vi "Joystick and Camera SHIH VP- external Connection.vi"(0 "Motion in":refnum<class "Motion.lvclass">, 1 "XYZTheta":dbl[](array[numeric]), 2 "Measurement Point":string, 3 "Inital GO":bool=TRUE) -> (7 "Motion out":refnum<class "Motion.lvclass">, 8 "Sum":dbl[](array[numeric]), 9 "Gantry":dbl[](array[numeric]), 10 "error out":errorcluster)   [LabVIEW 2016]
uses:
  Classes/Controllers/Motion/Copy of Motion Folder/Motion.lvclass
  Classes/Controllers/Camera/Copy of Camera Folder/Machine Vision.ctl
  Classes/Controllers/Camera/Copy of Camera Folder/Camera.lvclass
  Classes/Controllers/Camera/Copy of Controller Folder/Controller.lvclass
panel:
  in  "change move step":bool
  in  "step":dbl=15.0
  in  "Z go up":bool
  in  "Z go down":bool
  in  "Machine Vision":T1
  in  "object goes left":bool
  in  "object goes right":bool
  in  "object goes down":bool
  in  "object goes up":bool
  in  "Z go up 25 um":bool
  in  "Z go down 25 um":bool
  in  "Z go up 0.05 mm":bool
  in  "Z go down 0.05 mm":bool
  in  "Z go  up 0.1 mm":bool
  in  "Z go down 0.1 mm":bool
  in  "Machine Vision 2":T1=enum."None"
  out "Image 2":T2(plugin-control)
  out "Focus Index":dbl[](array[numeric])
  in  "interval":dbl=0.005
  out "Score":dbl[](array[numeric])
  out "Waveform Graph":dbl[](graph)
  in  "focus":bool
  out "Numeric":dbl
  in  "Go SUM":bool
  in  "Z Go":bool
  in  "Position":dbl
  in  "Go":bool
  in  "Joystick":bool
  in  "Stop":bool
  out "Image":T2(plugin-control)
  out "Camera":dbl[](array[numeric])
  # "0.1mm"
  # "0.01mm"
  # "um"
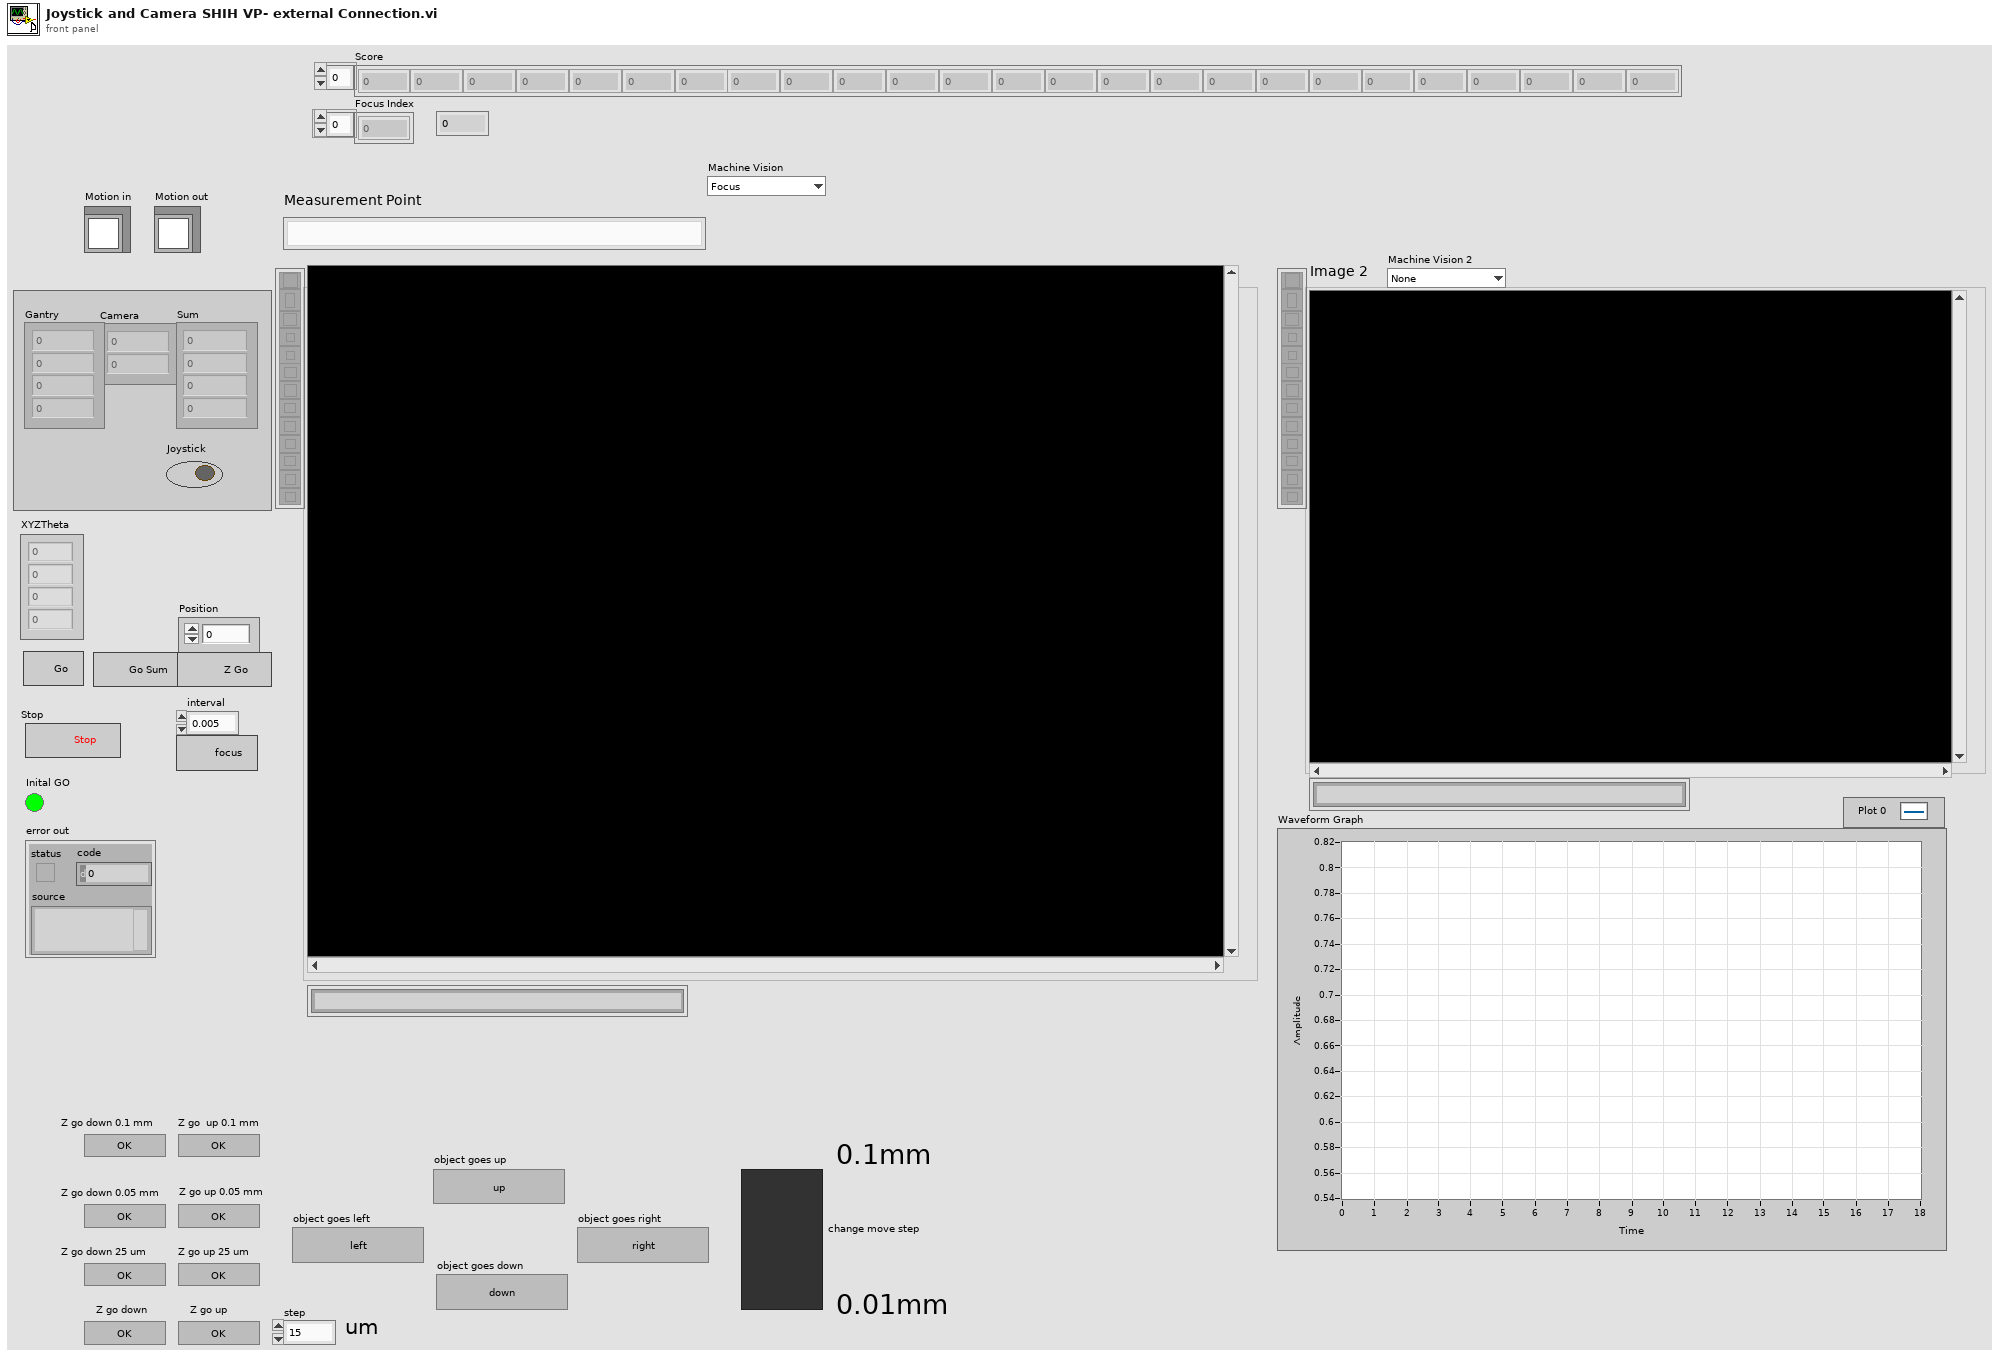
[diagram p1: front panel]
types:
  T1 = typedef "Camera.lvclass/Machine Vision.ctl" = enum16{"Focus", "chip cross", "LargeCircle", "None", "INTT HDI Mark", "INTT Sensor Cross", "INTT Chip Corner", "HPK Silicon", "circle"}
  T2 = typedef "IMAQ Image.ctl" = refnum<image>
  T3 = typedef "Controller.lvclass/Controllers.ctl" = cluster{"Copy of Motion.lvclass":refnum<class "Motion.lvclass">, "Copy of I-O.lvclass":refnum<class "I-O.lvclass">, "Copy of Dispenser.lvclass":refnum<class "Dispenser.lvclass">}
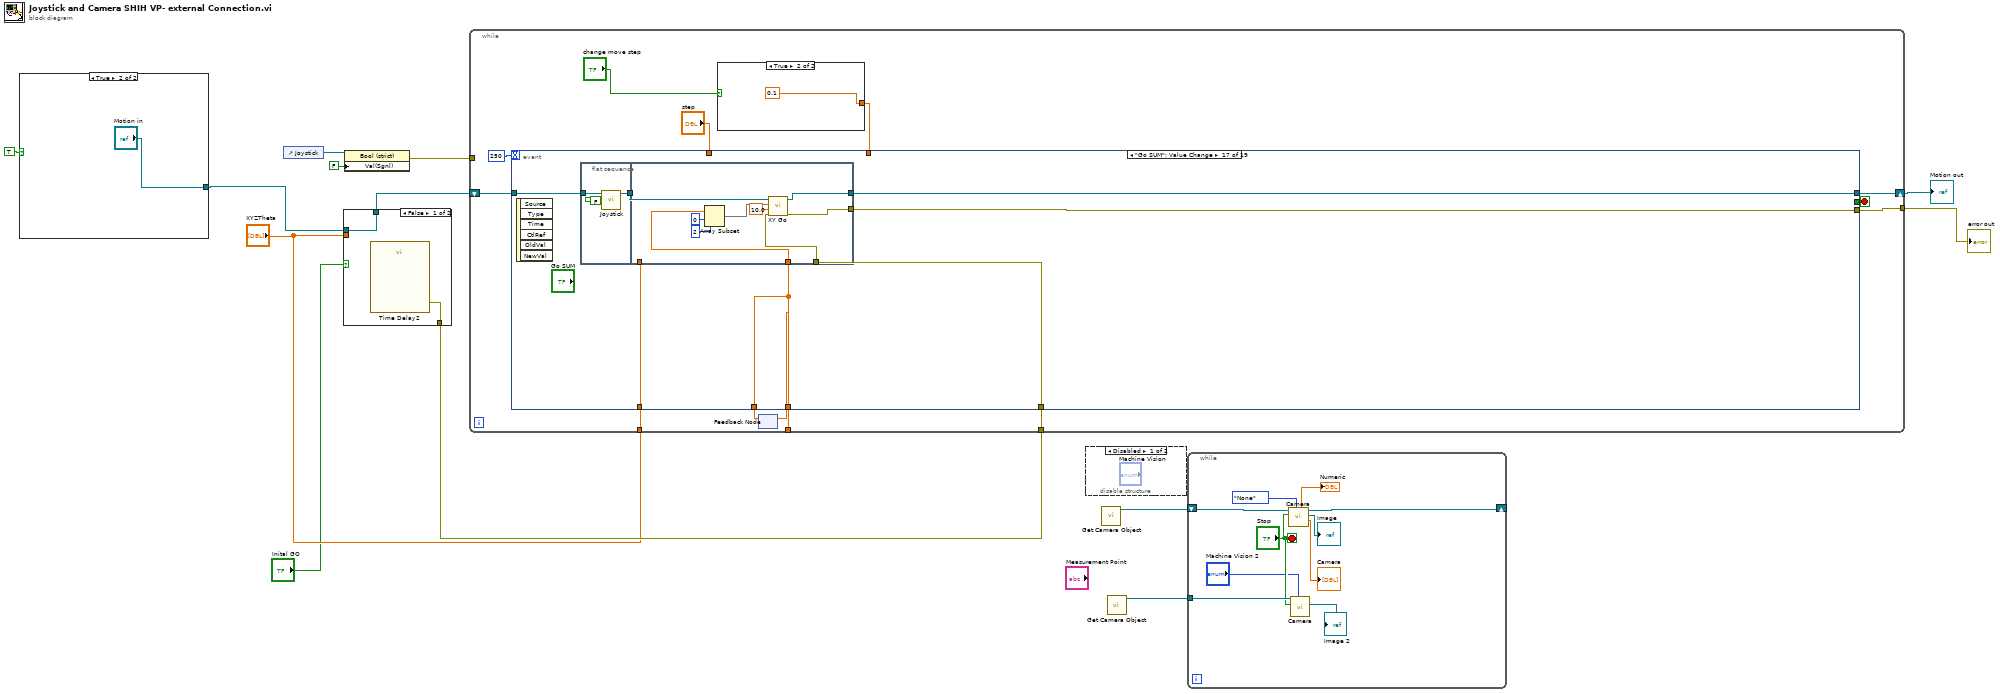
[diagram p0: block diagram]
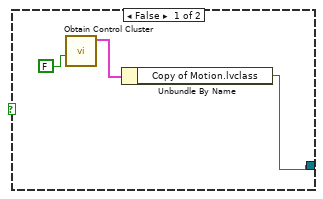
[diagram p3: hidden frame]
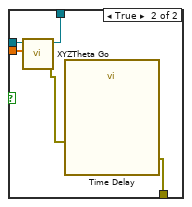
[diagram p4: hidden frame]
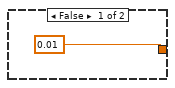
[diagram p5: hidden frame]
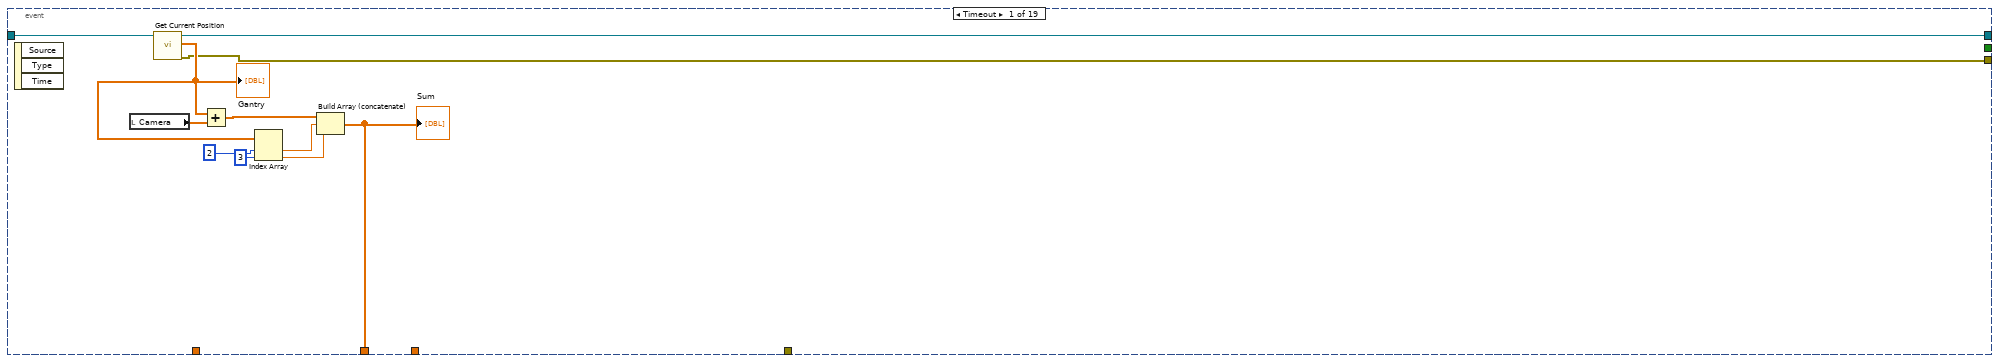
[diagram p6: hidden frame]
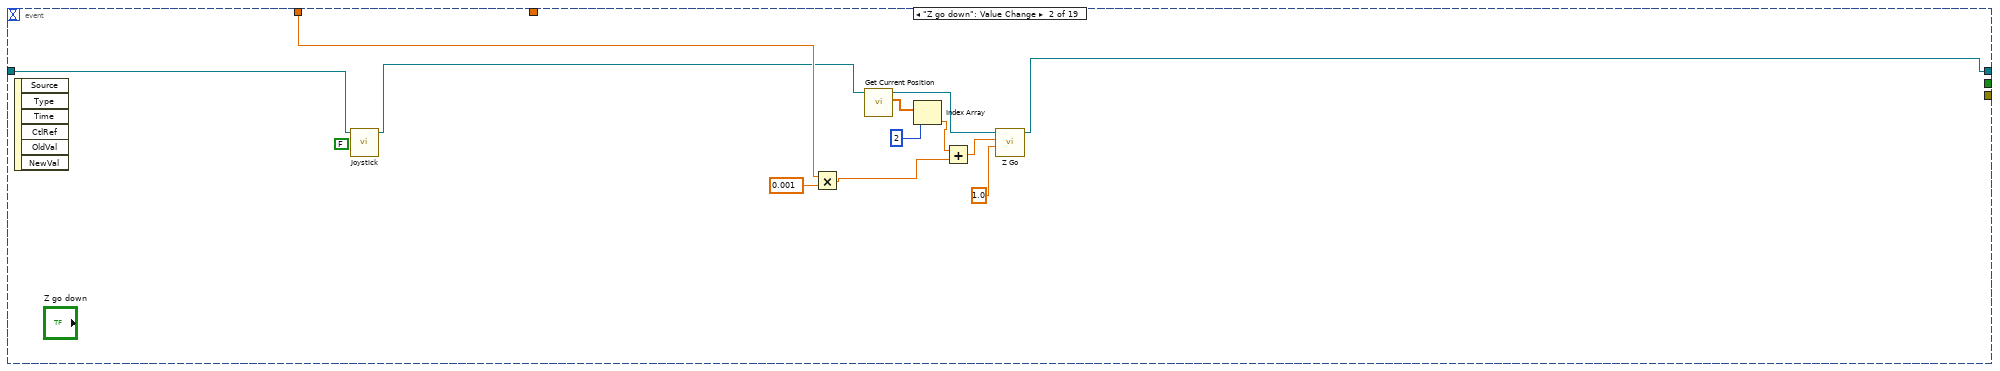
[diagram p7: hidden frame]
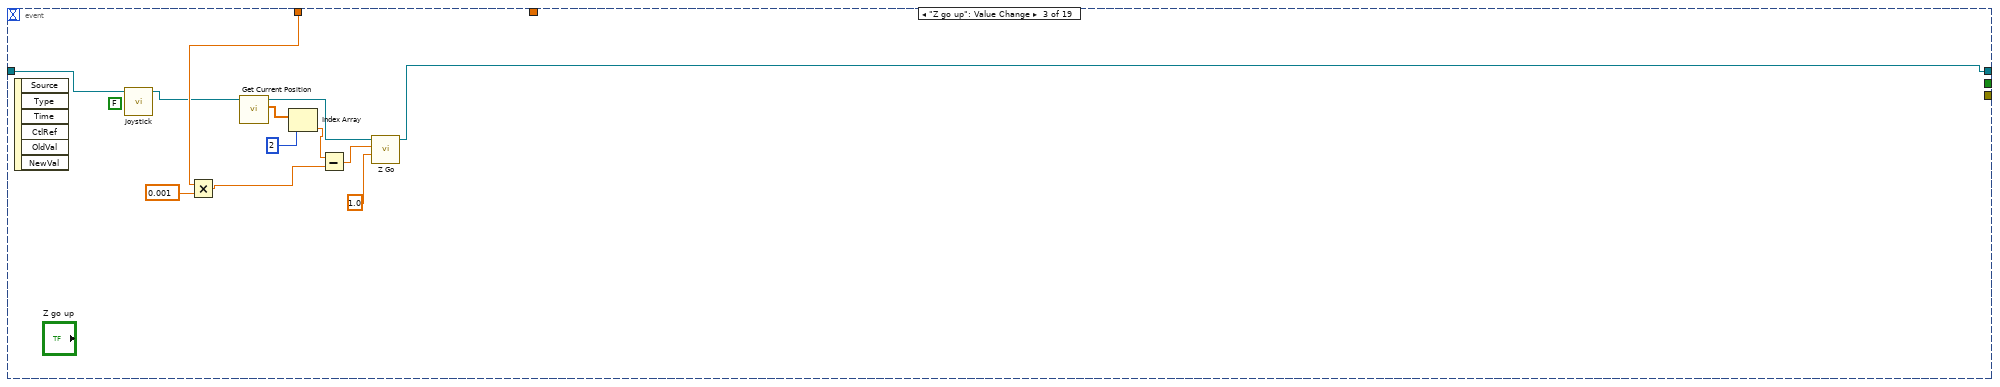
[diagram p8: hidden frame]
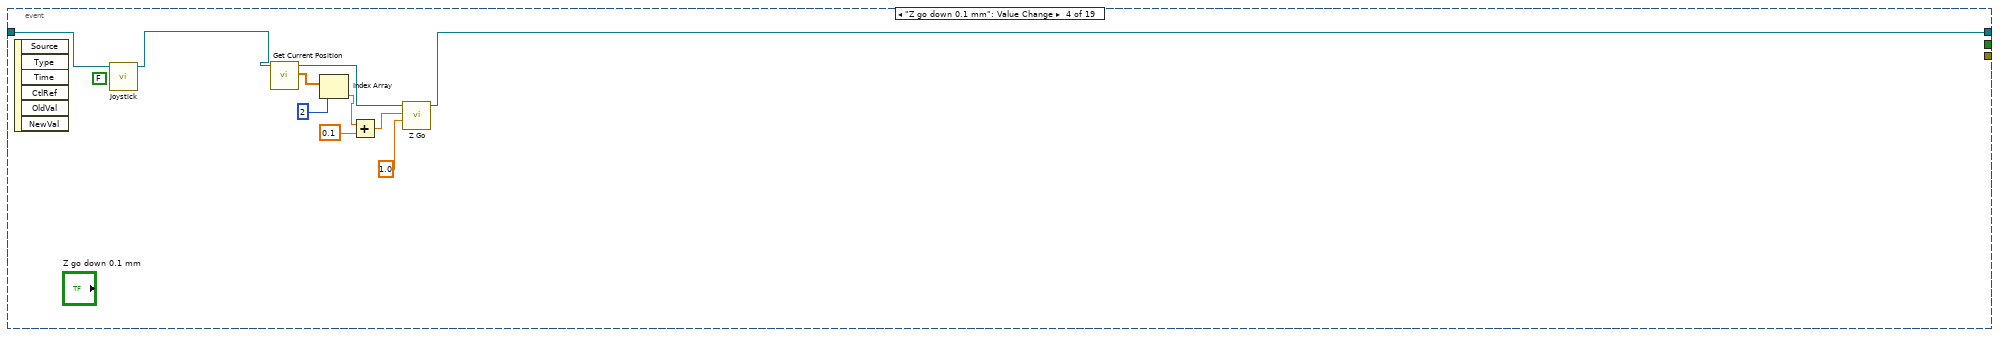
[diagram p9: hidden frame]
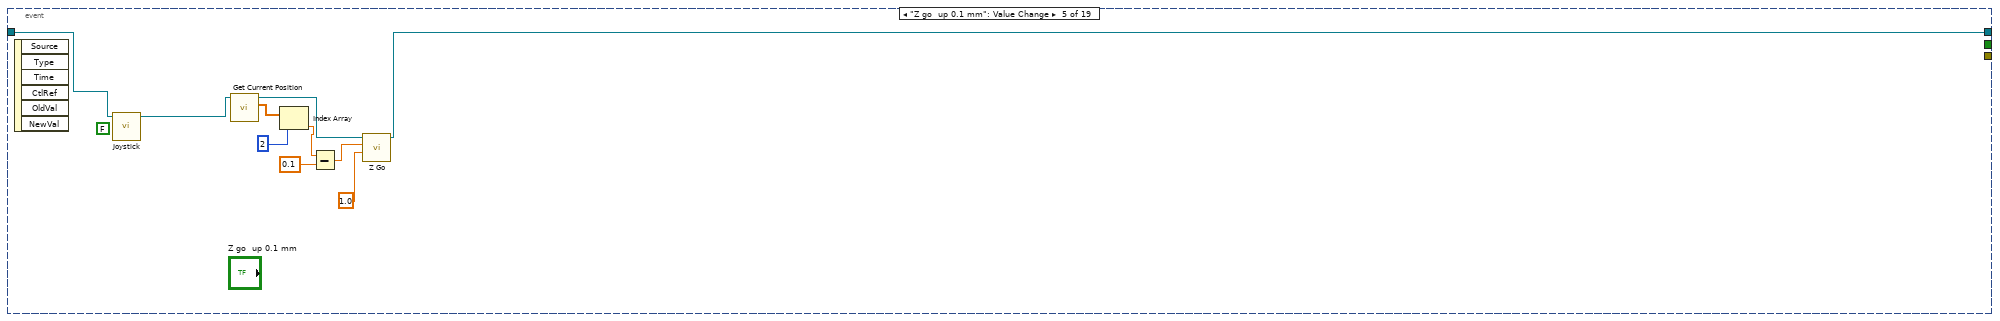
[diagram p10: hidden frame]
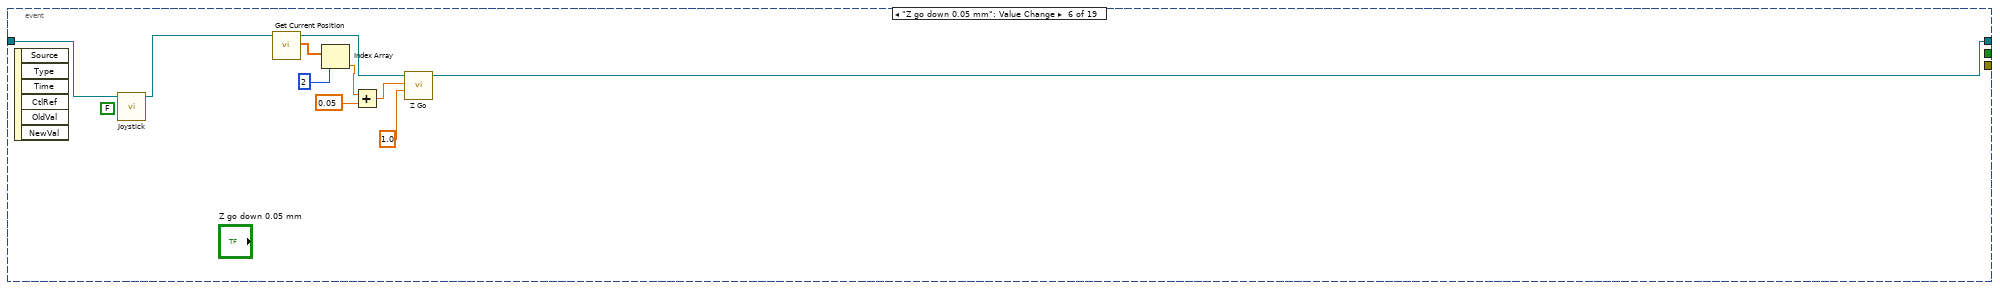
[diagram p11: hidden frame]
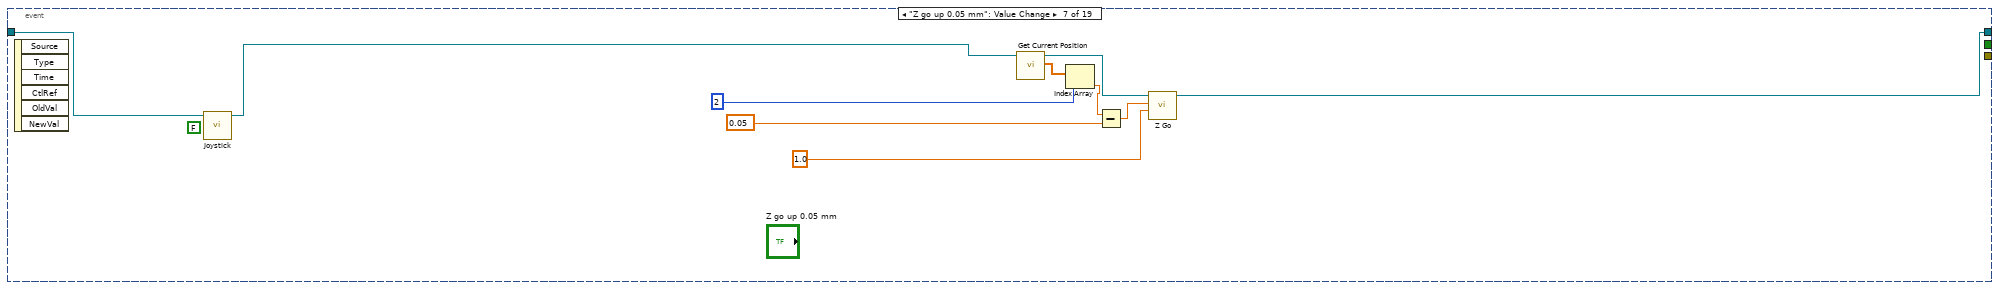
[diagram p12: hidden frame]
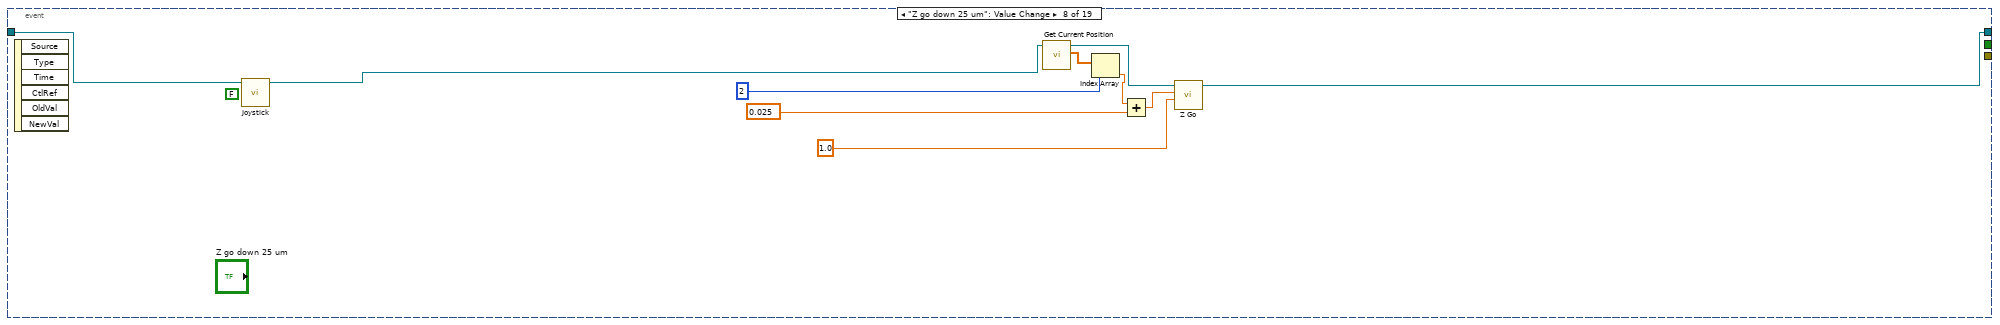
[diagram p13: hidden frame]
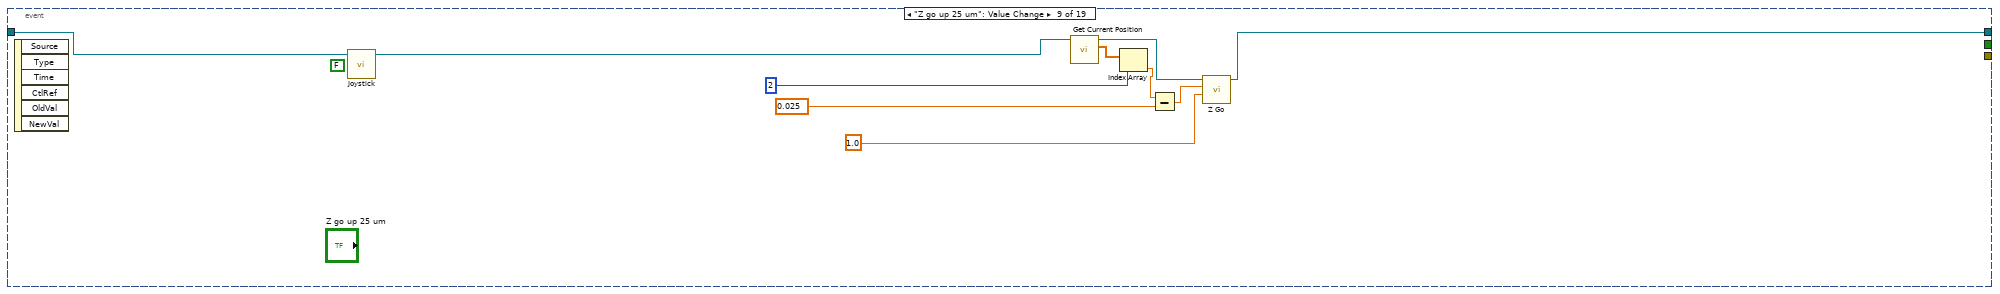
[diagram p14: hidden frame]
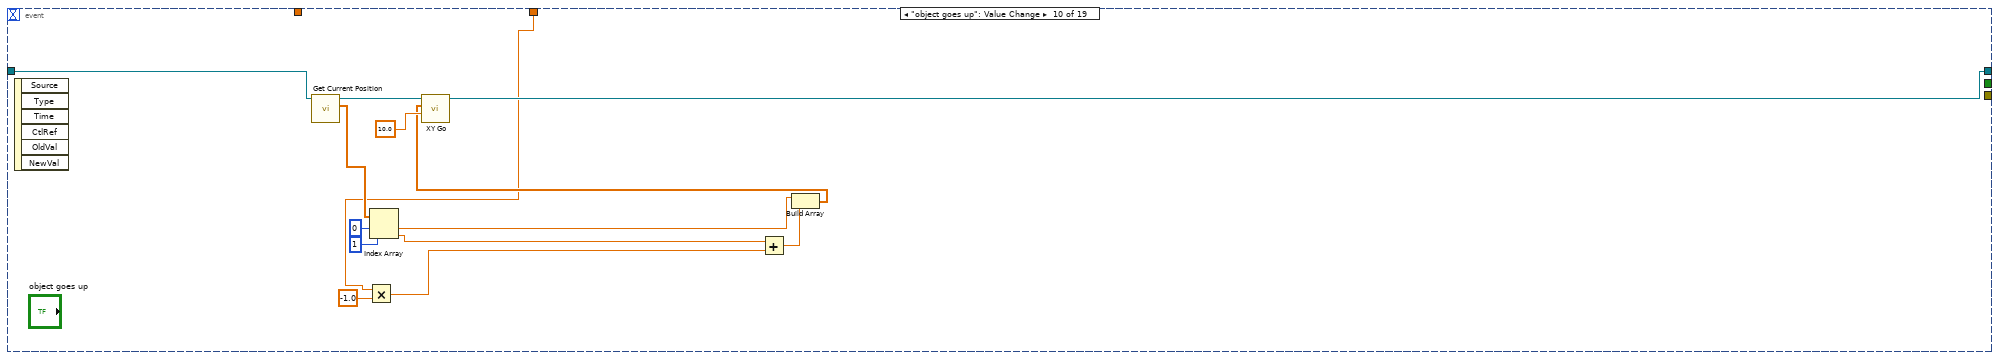
[diagram p15: hidden frame]
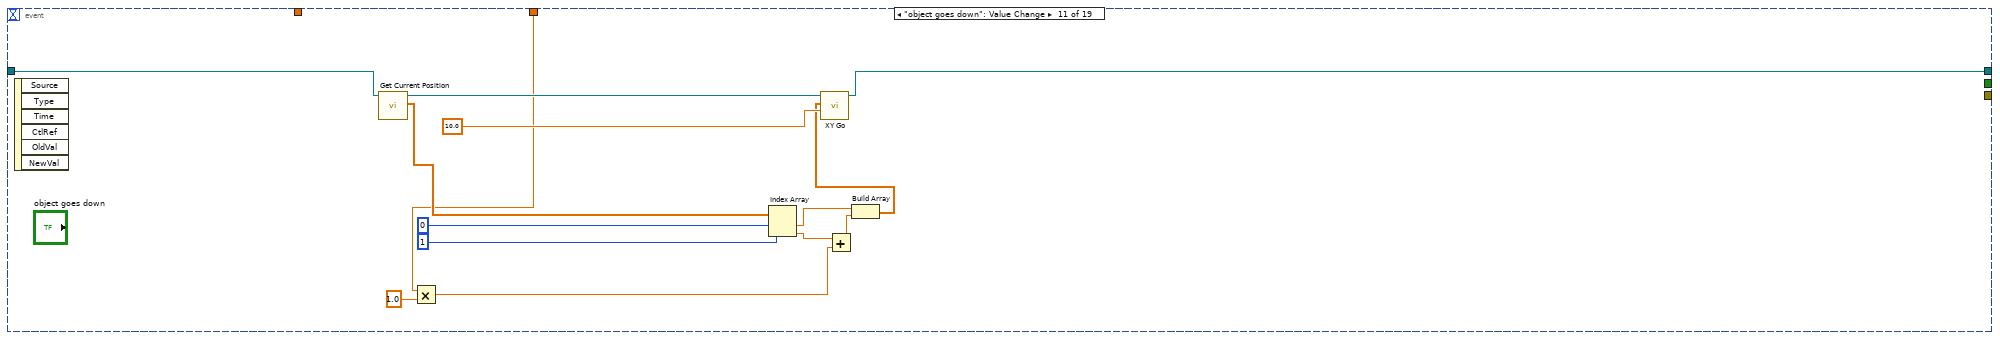
[diagram p16: hidden frame]
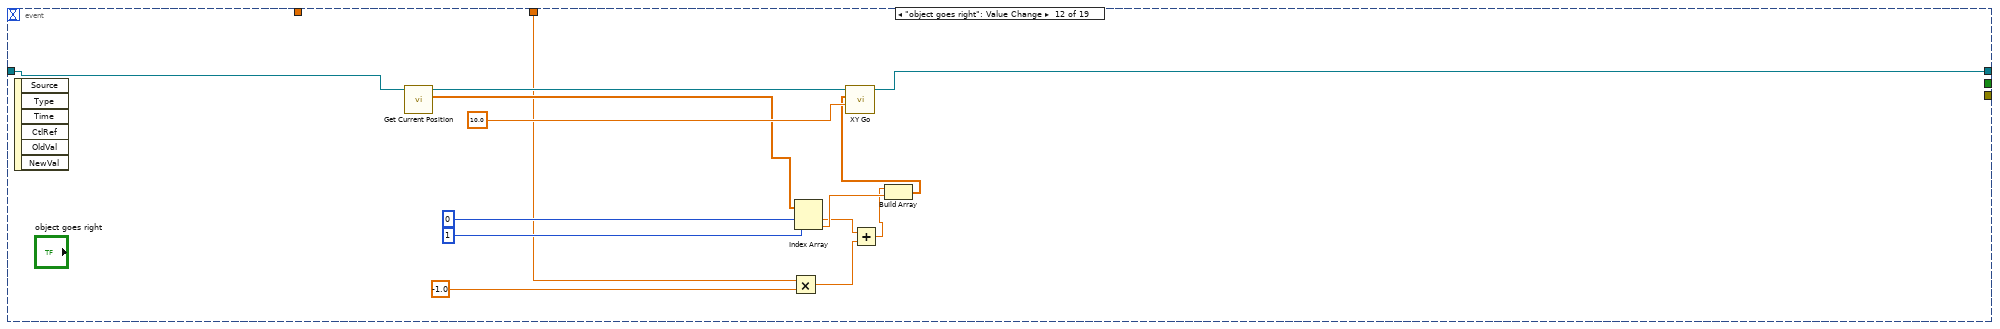
[diagram p17: hidden frame]
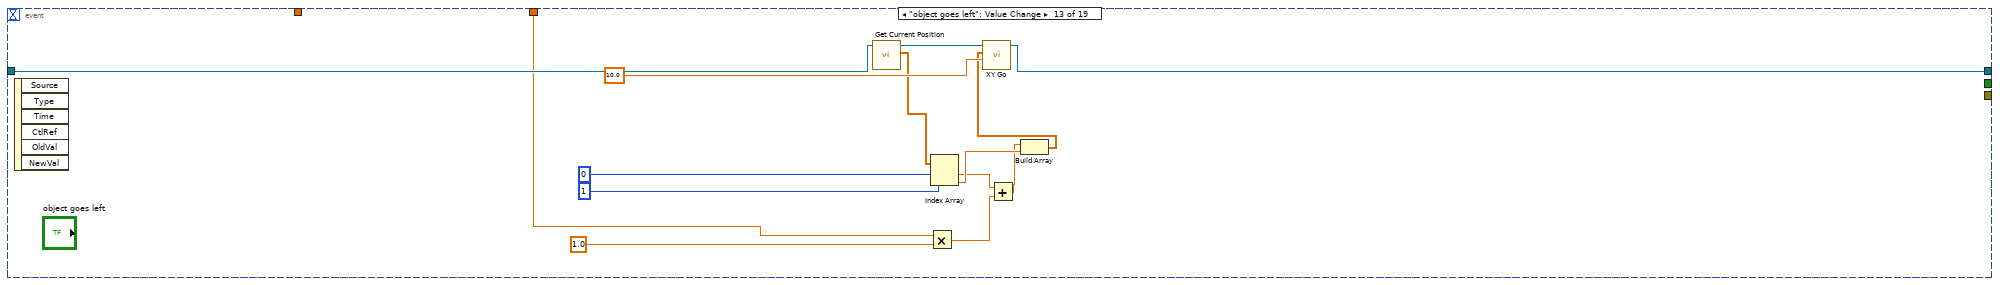
[diagram p18: hidden frame]
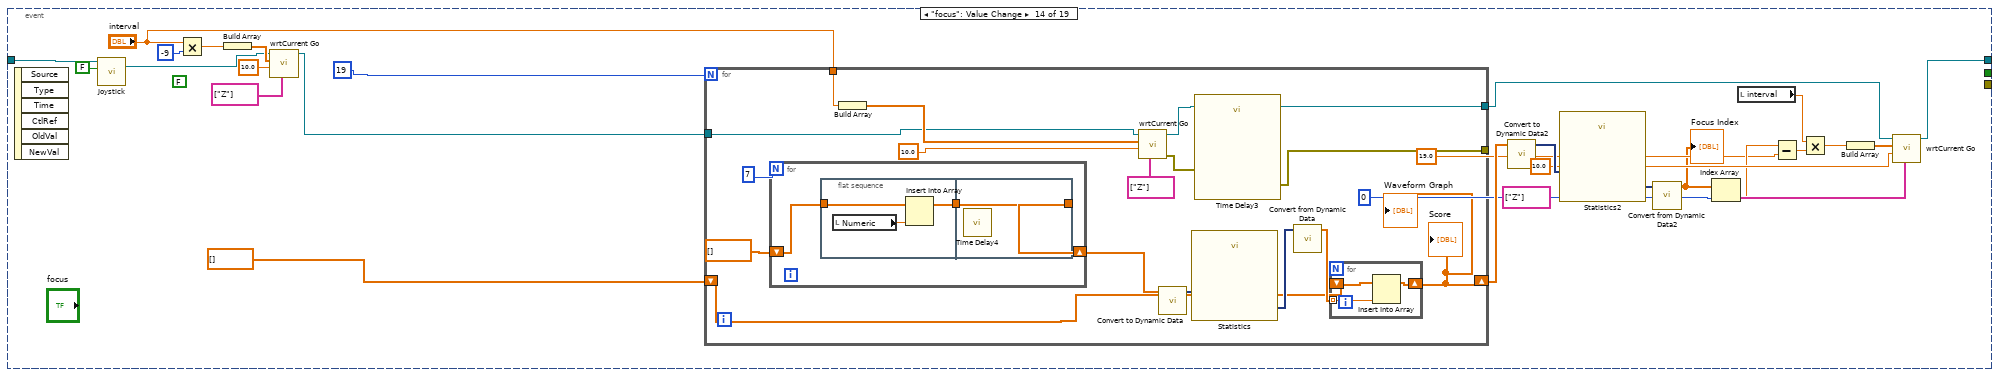
[diagram p19: hidden frame]
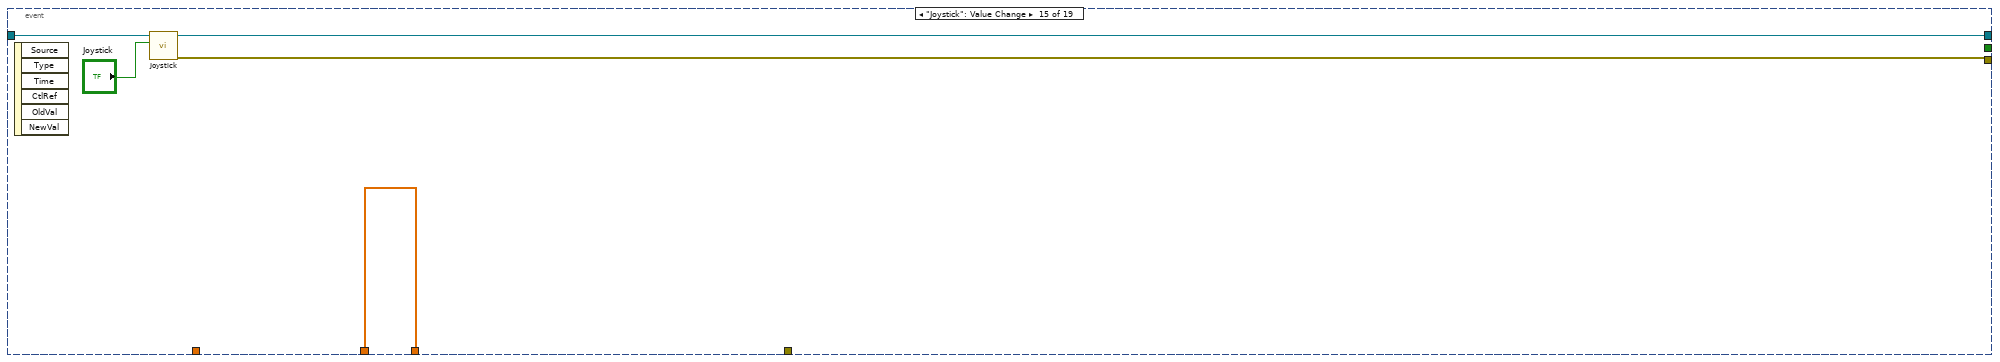
[diagram p20: hidden frame]
diagram:
  n1 = case shown="True" TRUE {
    tunnel: [w14 "Motion in"] -> w1
    frame False {
      n2 = call "Obtain Control Cluster.vi"("I/O"=FALSE) -> ("Control Out"=w16:T3)  [unwired: 10 in]
      n3 = Unbundle By Name(w16) -> ("Copy of Motion.lvclass"=w14:refnum<class "Motion.lvclass">)
    }
    frame True {
    }
  }
  n4 = control-ref of="Joystick"() -> (w12:refnum<vi>)
  n5 = case shown="False" "Inital GO" {
    tunnel: w1 -> [w19 w24]
    tunnel: [w19 w23] -> w7
    tunnel: [w18 w21] -> w6
    tunnel: "XYZTheta" -> [_ w20]
    frame False {
      n6 = call "Time Delay2"() -> ("error out"=w18:errorcluster)  [unwired: 11 in]
    }
    frame True {
      n7 = call "XYZTheta Go.vi"("XYZTheta In"=w20, "Motion in"=w24) -> ("error out"=w22:errorcluster, "Motion out"=w23:refnum<class "Motion.lvclass">)  [unwired: 7 in, 1 out]
      n8 = call "Time Delay"("error in (no error)"=w22) -> ("error out"=w21:errorcluster)  [unwired: 10 in]
    }
  }
  n9 = property class="Bool (strict)"(reference=w12, "Val(Sgnl)"=FALSE ("Value (Signaling)")) -> (error out=w11:errorcluster)  [unwired: 1 in, 1 out]
  n10 = while {
    shift-right: [w33] -> w9
    shift-left: w7 -> [w34]
    tunnel: w11 -> [_]
    tunnel: [w32] -> w8
    tunnel: w6 -> [w31]
    tunnel: "XYZTheta" -> [w30]
    tunnel: [w28] -> _
    stop <- w35 stop-if-true
    n11 = case shown="True" "change move step" {
      tunnel: [0.01 0.1] -> w25
      frame False {
      }
      frame True {
      }
    }
    n12 = feedback #1() -> (w28:dbl[])  [unwired: 1 in]
    n13 = event shown="[16] \"Go SUM\": Value Change" {
      selector: _ -> [_ _ _ _ _ _ _ _ _ _ _ _ _ _ _ _ _ _ _]
      dyn-events: _ -> [_ _ _ _ _ _ _ _ _ _ _ _ _ _ _ _ _ _ _]
      timeout: 250 -> [_ _ _ _ _ _ _ _ _ _ _ _ _ _ _ _ _ _ _]
      tunnel: [_ _ _ _ _ _ _ _ _ _ _ _ _ _ _ _ _ _ TRUE] -> w35
      tunnel: w34 -> [w48 w51 w63 w75 w85 w95 w105 w115 w125 w145 w155 w166 w180 w192 w247 w254 w279 w298 w302]
      tunnel: [w47 w52 w67 w76 w86 w96 w106 w116 w126 w144 w154 w167 w181 w191 w245 w253 w274 w297 w300] -> w33
      tunnel: [w42 _ _ _ _ _ _ _ _ _ _ _ _ _ w244 w251 w277 w292 _] -> w32
      tunnel: w31 -> [_ _ _ _ _ _ _ _ _ _ _ _ _ _ _ w250 w276 w293 _]
      tunnel: w30 -> [_ _ _ _ _ _ _ _ _ _ _ _ _ _ _ w249 w275 _ _]
      tunnel: [w39 _ _ _ _ _ _ _ _ _ _ _ _ _ w243 w248 w273 w294 w299] -> w29
      tunnel: w28 -> [_ _ _ _ _ _ _ _ _ _ _ _ _ _ w243 w248 w273 w294 w299]
      tunnel: "step" -> [_ w53 w65 _ _ _ _ _ _ _ _ _ _ _ _ _ _ _ _]
      tunnel: w25 -> [_ _ _ _ _ _ _ _ _ w134 w148 w162 w176 _ _ _ _ _ _]
      event Timeout {
        n14 = event-data() -> ()  [unwired: 1 in, 3 out]
        n15 = local read "Camera"() -> (w49:dbl[])
        n16 = call-dynamic "Get Current Position.vi"("Motion in"=w48) -> ("error out"=w42:errorcluster, "XYZTheta Out"=w45:dbl[], "Motion out"=w47:refnum<class "Motion.lvclass">)  [unwired: 8 in]
        "Gantry" <- w45
        n17 = Add(x=w45, y=w49) -> (x+y=w46:dbl[])
        n18 = Index Array(array=w45, index #1=2 ("index"), index #2=3 ("index")) -> (element #1=w43:dbl, element #2=w40:dbl)
        n19 = Build Array (concatenate)(w46, w43, w40) -> (w39:dbl[])
        "Sum" <- w39
      }
      event "Z go down": Value Change {
        (unwired) FALSE ("Joystick")
        n20 = event-data() -> ()  [unwired: 1 in, 6 out]
        n21 = call-dynamic "Joystick.vi"("Motion in"=w51) -> ("Motion out"=w50:refnum<class "Motion.lvclass">)  [unwired: 9 in, 1 out]
        n22 = Multiply(x=w53, y=0.001) -> (x*y=w55:dbl)
        n23 = call-dynamic "Get Current Position.vi"("Motion in"=w50) -> ("XYZTheta Out"=w61:dbl[], "Motion out"=w59:refnum<class "Motion.lvclass">)  [unwired: 8 in, 1 out]
        n24 = Index Array(array=w61, index=2) -> (element=w56:dbl)
        n25 = Add(x=w56, y=w55) -> (x+y=w57:dbl)
        n26 = call-dynamic "Z Go.vi"("Speed"=1.0, "Position"=w57, "Motion in"=w59) -> ("Motion out"=w52:refnum<class "Motion.lvclass">)  [unwired: 7 in, 1 out]
      }
      event "Z go up": Value Change {
        (unwired) FALSE ("Joystick")
        n27 = event-data() -> ()  [unwired: 1 in, 6 out]
        n28 = call-dynamic "Joystick.vi"("Motion in"=w63) -> ("Motion out"=w62:refnum<class "Motion.lvclass">)  [unwired: 9 in, 1 out]
        n29 = Multiply(x=w65, y=0.001) -> (x*y=w66:dbl)
        n30 = call-dynamic "Get Current Position.vi"("Motion in"=w62) -> ("XYZTheta Out"=w73:dbl[], "Motion out"=w71:refnum<class "Motion.lvclass">)  [unwired: 8 in, 1 out]
        n31 = Index Array(array=w73, index=2) -> (element=w68:dbl)
        n32 = Subtract(x=w68, y=w66) -> (x-y=w69:dbl)
        n33 = call-dynamic "Z Go.vi"("Speed"=1.0, "Position"=w69, "Motion in"=w71) -> ("Motion out"=w67:refnum<class "Motion.lvclass">)  [unwired: 7 in, 1 out]
      }
      event "Z go down 0.1 mm": Value Change {
        (unwired) FALSE ("Joystick")
        n34 = event-data() -> ()  [unwired: 1 in, 6 out]
        n35 = call-dynamic "Joystick.vi"("Motion in"=w75) -> ("Motion out"=w74:refnum<class "Motion.lvclass">)  [unwired: 9 in, 1 out]
        n36 = call-dynamic "Get Current Position.vi"("Motion in"=w74) -> ("XYZTheta Out"=w83:dbl[], "Motion out"=w81:refnum<class "Motion.lvclass">)  [unwired: 8 in, 1 out]
        n37 = Index Array(array=w83, index=2) -> (element=w78:dbl)
        n38 = Add(x=w78, y=0.1) -> (x+y=w79:dbl)
        n39 = call-dynamic "Z Go.vi"("Speed"=1.0, "Position"=w79, "Motion in"=w81) -> ("Motion out"=w76:refnum<class "Motion.lvclass">)  [unwired: 7 in, 1 out]
      }
      event "Z go  up 0.1 mm": Value Change {
        (unwired) FALSE ("Joystick")
        n40 = event-data() -> ()  [unwired: 1 in, 6 out]
        n41 = call-dynamic "Joystick.vi"("Motion in"=w85) -> ("Motion out"=w84:refnum<class "Motion.lvclass">)  [unwired: 9 in, 1 out]
        n42 = call-dynamic "Get Current Position.vi"("Motion in"=w84) -> ("XYZTheta Out"=w93:dbl[], "Motion out"=w91:refnum<class "Motion.lvclass">)  [unwired: 8 in, 1 out]
        n43 = Index Array(array=w93, index=2) -> (element=w88:dbl)
        n44 = Subtract(x=w88, y=0.1) -> (x-y=w89:dbl)
        n45 = call-dynamic "Z Go.vi"("Speed"=1.0, "Position"=w89, "Motion in"=w91) -> ("Motion out"=w86:refnum<class "Motion.lvclass">)  [unwired: 7 in, 1 out]
      }
      event "Z go down 0.05 mm": Value Change {
        (unwired) FALSE ("Joystick")
        n46 = event-data() -> ()  [unwired: 1 in, 6 out]
        n47 = call-dynamic "Joystick.vi"("Motion in"=w95) -> ("Motion out"=w94:refnum<class "Motion.lvclass">)  [unwired: 9 in, 1 out]
        n48 = call-dynamic "Get Current Position.vi"("Motion in"=w94) -> ("XYZTheta Out"=w103:dbl[], "Motion out"=w101:refnum<class "Motion.lvclass">)  [unwired: 8 in, 1 out]
        n49 = Index Array(array=w103, index=2) -> (element=w98:dbl)
        n50 = Add(x=w98, y=0.05) -> (x+y=w99:dbl)
        n51 = call-dynamic "Z Go.vi"("Speed"=1.0, "Position"=w99, "Motion in"=w101) -> ("Motion out"=w96:refnum<class "Motion.lvclass">)  [unwired: 7 in, 1 out]
      }
      event "Z go up 0.05 mm": Value Change {
        (unwired) FALSE ("Joystick")
        n52 = event-data() -> ()  [unwired: 1 in, 6 out]
        n53 = call-dynamic "Joystick.vi"("Motion in"=w105) -> ("Motion out"=w104:refnum<class "Motion.lvclass">)  [unwired: 9 in, 1 out]
        n54 = call-dynamic "Get Current Position.vi"("Motion in"=w104) -> ("XYZTheta Out"=w113:dbl[], "Motion out"=w111:refnum<class "Motion.lvclass">)  [unwired: 8 in, 1 out]
        n55 = Index Array(array=w113, index=2) -> (element=w108:dbl)
        n56 = Subtract(x=w108, y=0.05) -> (x-y=w109:dbl)
        n57 = call-dynamic "Z Go.vi"("Speed"=1.0, "Position"=w109, "Motion in"=w111) -> ("Motion out"=w106:refnum<class "Motion.lvclass">)  [unwired: 7 in, 1 out]
      }
      event "Z go down 25 um": Value Change {
        (unwired) FALSE ("Joystick")
        n58 = event-data() -> ()  [unwired: 1 in, 6 out]
        n59 = call-dynamic "Joystick.vi"("Motion in"=w115) -> ("Motion out"=w114:refnum<class "Motion.lvclass">)  [unwired: 9 in, 1 out]
        n60 = call-dynamic "Get Current Position.vi"("Motion in"=w114) -> ("XYZTheta Out"=w123:dbl[], "Motion out"=w121:refnum<class "Motion.lvclass">)  [unwired: 8 in, 1 out]
        n61 = Index Array(array=w123, index=2) -> (element=w118:dbl)
        n62 = Add(x=w118, y=0.025) -> (x+y=w119:dbl)
        n63 = call-dynamic "Z Go.vi"("Speed"=1.0, "Position"=w119, "Motion in"=w121) -> ("Motion out"=w116:refnum<class "Motion.lvclass">)  [unwired: 7 in, 1 out]
      }
      event "Z go up 25 um": Value Change {
        (unwired) FALSE ("Joystick")
        n64 = event-data() -> ()  [unwired: 1 in, 6 out]
        n65 = call-dynamic "Joystick.vi"("Motion in"=w125) -> ("Motion out"=w124:refnum<class "Motion.lvclass">)  [unwired: 9 in, 1 out]
        n66 = call-dynamic "Get Current Position.vi"("Motion in"=w124) -> ("XYZTheta Out"=w133:dbl[], "Motion out"=w131:refnum<class "Motion.lvclass">)  [unwired: 8 in, 1 out]
        n67 = Index Array(array=w133, index=2) -> (element=w128:dbl)
        n68 = Subtract(x=w128, y=0.025) -> (x-y=w129:dbl)
        n69 = call-dynamic "Z Go.vi"("Speed"=1.0, "Position"=w129, "Motion in"=w131) -> ("Motion out"=w126:refnum<class "Motion.lvclass">)  [unwired: 7 in, 1 out]
      }
      event "object goes up": Value Change {
        n70 = event-data() -> ()  [unwired: 1 in, 6 out]
        n71 = call-dynamic "Get Current Position.vi"("Motion in"=w145) -> ("XYZTheta Out"=w143:dbl[], "Motion out"=w147:refnum<class "Motion.lvclass">)  [unwired: 8 in, 1 out]
        n72 = Multiply(x=w134, y=-1.0) -> (x*y=w139:dbl)
        n73 = Index Array(array=w143, index #1=0 ("index"), index #2=1 ("index")) -> (element #1=w137:dbl, element #2=w136:dbl)
        n74 = Add(x=w136, y=w139) -> (x+y=w135:dbl)
        n75 = Build Array(w137, w135) -> (w140:dbl[])
        n76 = call-dynamic "XY Go.vi"("Speed"=10.0, "XY"=w140, "Motion in"=w147) -> ("Motion out"=w144:refnum<class "Motion.lvclass">)  [unwired: 7 in, 1 out]
      }
      event "object goes down": Value Change {
        n77 = event-data() -> ()  [unwired: 1 in, 6 out]
        n78 = call-dynamic "Get Current Position.vi"("Motion in"=w155) -> ("XYZTheta Out"=w159:dbl[], "Motion out"=w161:refnum<class "Motion.lvclass">)  [unwired: 8 in, 1 out]
        n79 = Multiply(x=w148, y=1.0) -> (x*y=w153:dbl)
        n80 = Index Array(array=w159, index #1=0 ("index"), index #2=1 ("index")) -> (element #1=w151:dbl, element #2=w150:dbl)
        n81 = Add(x=w150, y=w153) -> (x+y=w149:dbl)
        n82 = Build Array(w151, w149) -> (w156:dbl[])
        n83 = call-dynamic "XY Go.vi"("Speed"=10.0, "XY"=w156, "Motion in"=w161) -> ("Motion out"=w154:refnum<class "Motion.lvclass">)  [unwired: 7 in, 1 out]
      }
      event "object goes right": Value Change {
        n84 = event-data() -> ()  [unwired: 1 in, 6 out]
        n85 = call-dynamic "Get Current Position.vi"("Motion in"=w166) -> ("XYZTheta Out"=w173:dbl[], "Motion out"=w175:refnum<class "Motion.lvclass">)  [unwired: 8 in, 1 out]
        n86 = Multiply(x=w162, y=-1.0) -> (x*y=w169:dbl)
        n87 = Index Array(array=w173, index #1=0 ("index"), index #2=1 ("index")) -> (element #1=w164:dbl, element #2=w165:dbl)
        n88 = Add(x=w164, y=w169) -> (x+y=w163:dbl)
        n89 = Build Array(w163, w165) -> (w170:dbl[])
        n90 = call-dynamic "XY Go.vi"("Speed"=10.0, "XY"=w170, "Motion in"=w175) -> ("Motion out"=w167:refnum<class "Motion.lvclass">)  [unwired: 7 in, 1 out]
      }
      event "object goes left": Value Change {
        n91 = event-data() -> ()  [unwired: 1 in, 6 out]
        n92 = call-dynamic "Get Current Position.vi"("Motion in"=w180) -> ("XYZTheta Out"=w187:dbl[], "Motion out"=w189:refnum<class "Motion.lvclass">)  [unwired: 8 in, 1 out]
        n93 = Multiply(x=w176, y=1.0) -> (x*y=w183:dbl)
        n94 = Index Array(array=w187, index #1=0 ("index"), index #2=1 ("index")) -> (element #1=w178:dbl, element #2=w179:dbl)
        n95 = Add(x=w178, y=w183) -> (x+y=w177:dbl)
        n96 = Build Array(w177, w179) -> (w184:dbl[])
        n97 = call-dynamic "XY Go.vi"("Speed"=10.0, "XY"=w184, "Motion in"=w189) -> ("Motion out"=w181:refnum<class "Motion.lvclass">)  [unwired: 7 in, 1 out]
      }
      event "focus": Value Change {
        (unwired) FALSE ("Joystick")
        n98 = event-data() -> ()  [unwired: 1 in, 6 out]
        n99 = call-dynamic "Joystick.vi"("Joystick"=FALSE, "Motion in"=w192) -> ("Motion out"=w194:refnum<class "Motion.lvclass">)  [unwired: 8 in, 1 out]
        n100 = Multiply(x="interval", y=-9) -> (x*y=w209:dbl)
        n101 = Build Array(w209) -> (w211:dbl[])
        n102 = call-dynamic "wrtCurrent Go.vi"("axis names"=string[] ["Z"] ("Axis"), "Speed"=10.0, "distances"=w211, "Motion in"=w194) -> ("Motion out"=w215:refnum<class "Motion.lvclass">)  [unwired: 6 in, 1 out]
        n103 = for {
          N: 19 -> [_]
          tunnel: w215 -> [w217]
          tunnel: [w221] -> w201
          shift-right: [w218] -> w207
          shift-left: dbl[] [] -> [w219]
          tunnel: "interval" -> [w224]
          tunnel: [w220] -> _
          n104 = for {
            N: 7 -> [_]
            shift-right: [w238] -> w229
            shift-left: dbl[] [] -> [w237]
            n105 = flat-sequence {
              tunnel: w237 -> [w240]
              tunnel: [w241] -> w236
              tunnel: [w242] -> w238
              tunnel: w236 -> [w242]
              frame #0 {
                n106 = local read "Numeric"() -> (w239:dbl)
                n107 = Insert Into Array(array=w240, new element=w239) -> (w241:dbl[])  [unwired: 1 in]
              }
              frame #1 {
                n108 = call "Time Delay4"() -> ()  [unwired: 11 in, 1 out]
              }
            }
          }
          n109 = Build Array(w224) -> (w223:dbl[])
          n110 = call-dynamic "wrtCurrent Go.vi"("axis names"=string[] ["Z"] ("Axis"), "Speed"=10.0, "distances"=w223, "Motion in"=w217) -> ("error out"=w230:errorcluster, "Motion out"=w221:refnum<class "Motion.lvclass">)  [unwired: 6 in]
          n111 = call "Convert to Dynamic Data"("Array"=w229) -> ("Dynamic Data Type"=w228:dynamicdata)  [unwired: 3 in]
          n112 = call "Statistics"("Signals"=w228) -> ("Arithmetic Mean"=w226:dynamicdata)  [unwired: 25 in, 1 out]
          n113 = call "Time Delay3"("error in (no error)"=w230) -> ("error out"=w220:errorcluster)  [unwired: 10 in]
          n114 = call "Convert from Dynamic Data"("Dynamic Data Type"=w226) -> ("Array"=w222:dbl[])  [unwired: 3 in]
          n115 = for {
            tunnel: w222 -> [w235] mode=indexing
            shift-right: [w234] -> w218
            shift-left: w219 -> [w233]
            n116 = Insert Into Array(array=w233, new element=w235) -> (w234:dbl[])  [unwired: 1 in]
          }
          "Score" <- w218
          "Waveform Graph" <- w218
        }
        n117 = call "Convert to Dynamic Data2"("Array"=w207) -> ("Dynamic Data Type"=w206:dynamicdata)  [unwired: 3 in]
        n118 = call "Statistics2"("Signals"=w206) -> ("Index of Max"=w205:dynamicdata)  [unwired: 25 in, 1 out]
        n119 = call "Convert from Dynamic Data2"("Dynamic Data Type"=w205) -> ("Array"=w193:dbl[])  [unwired: 3 in]
        "Focus Index" <- w193
        n120 = Index Array(array=w193, index=0) -> (element=w196:dbl)
        n121 = local read "interval"() -> (w199:dbl)
        n122 = Subtract(x=w196, y=19.0 ("x")) -> (x-y=w200:dbl)
        n123 = Multiply(x=w199, y=w200) -> (x*y=w198:dbl)
        n124 = Build Array(w198) -> (w197:dbl[])
        n125 = call-dynamic "wrtCurrent Go.vi"("axis names"=string[] ["Z"] ("Axis"), "Speed"=10.0, "distances"=w197, "Motion in"=w201) -> ("Motion out"=w191:refnum<class "Motion.lvclass">)  [unwired: 6 in, 1 out]
      }
      event "Joystick": Value Change {
        n126 = event-data() -> ()  [unwired: 1 in, 6 out]
        n127 = call-dynamic "Joystick.vi"("Joystick"="Joystick", "Motion in"=w247) -> ("error out"=w244:errorcluster, "Motion out"=w245:refnum<class "Motion.lvclass">)  [unwired: 8 in]
      }
      event "Go": Value Change {
        n128 = event-data() -> ()  [unwired: 1 in, 6 out]
        n129 = flat-sequence {
          tunnel: w254 -> [w256]
          tunnel: [w255] -> w252
          tunnel: [w261] -> w253
          tunnel: w252 -> [w264]
          tunnel: [w260] -> w251
          tunnel: w250 -> [w259]
          tunnel: w249 -> [w258]
          frame #0 {
            n130 = call-dynamic "Joystick.vi"("Joystick"=FALSE, "Motion in"=w256) -> ("Motion out"=w255:refnum<class "Motion.lvclass">)  [unwired: 8 in, 1 out]
          }
          frame #1 {
            n131 = for {
              tunnel: w258 -> [w270] mode=indexing
              tunnel: [w268] -> w263 mode=indexing
              shift-right: [w266] -> w262
              shift-left: w264 -> [w267]
              i -> [w272]
              n132 = Equal To 0?(x=w270) -> (x = 0?=w271:bool)
              n133 = call-dynamic "Get Current Position.vi"("Motion in"=w267) -> ("XYZTheta Out"=w265:dbl[], "Motion out"=w266:refnum<class "Motion.lvclass">)  [unwired: 8 in, 1 out]
              n134 = Index Array(array=w265, index=w272) -> (element=w269:dbl)
              n135 = Select(t=w269, s=w271, f=w270) -> (s? t:f=w268:dbl)
            }
            n136 = call "XYZTheta Go.vi"("error in (no error)"=w259, "XYZTheta In"=w263, "Motion in"=w262) -> ("error out"=w260:errorcluster, "Motion out"=w261:refnum<class "Motion.lvclass">)  [unwired: 6 in, 1 out]
          }
        }
      }
      event "Go SUM": Value Change {
        n137 = event-data() -> ()  [unwired: 1 in, 6 out]
        n138 = flat-sequence {
          tunnel: w279 -> [w281]
          tunnel: [w280] -> w278
          tunnel: w278 -> [w287]
          tunnel: [w285] -> w277
          tunnel: w276 -> [w286]
          tunnel: w275 -> [_]
          tunnel: w273 -> [w290]
          tunnel: [w284] -> w274
          frame #0 {
            n139 = call-dynamic "Joystick.vi"("Joystick"=FALSE, "Motion in"=w281) -> ("Motion out"=w280:refnum<class "Motion.lvclass">)  [unwired: 8 in, 1 out]
          }
          frame #1 {
            n140 = Array Subset(array=w290, index=0, length=2) -> (w283:dbl[])
            n141 = call-dynamic "XY Go.vi"("error in (no error)"=w286, "Speed"=10.0, "XY"=w283, "Motion in"=w287) -> ("error out"=w285:errorcluster, "Motion out"=w284:refnum<class "Motion.lvclass">)  [unwired: 6 in]
          }
        }
      }
      event "Z Go": Value Change {
        n142 = event-data() -> ()  [unwired: 1 in, 6 out]
        n143 = call-dynamic "Z Go.vi"("error in (no error)"=w293, "Speed"=2.0, "Position"="Position", "Motion in"=w298) -> ("error out"=w292:errorcluster, "Motion out"=w297:refnum<class "Motion.lvclass">)  [unwired: 6 in]
      }
      event "Stop": Value Change {
        n144 = event-data() -> ()  [unwired: 1 in, 5 out]
        n145 = call-dynamic "Joystick.vi"("Joystick"=FALSE, "Motion in"=w302) -> ("Motion out"=w300:refnum<class "Motion.lvclass">)  [unwired: 8 in, 1 out]
      }
    }
    n146 = feedback-in #1(w29) -> ()
  }
  "error out" <- w8
  "Motion out" <- w9
  n147 = disable-structure shown="Disabled" {
    frame Disabled {
    }
    frame Enabled {
    }
  }
  n148 = call "Get Camera Object.vi"() -> ("Camera out"=w10:refnum<class "Camera.lvclass">)  [unwired: 10 in, 1 out]
  n149 = call "Get Camera Object.vi"() -> ("Camera out"=w3:refnum<class "Camera.lvclass">)  [unwired: 10 in, 1 out]
  n150 = while {
    shift-right: [w312] -> _
    shift-left: w10 -> [w313]
    tunnel: w3 -> [w308]
    stop <- "Stop" stop-if-true
    n151 = call "Camera.vi"("Machine Vision"=Machine_Vision."None", "Stop"="Stop", "Camera in"=w313) -> ("Camera"=→"Camera":dbl[], "Image"=→"Image":T2, "Camera out"=w312:refnum<class "Camera.lvclass">, "Numeric"=→"Numeric":dbl)  [unwired: 2 in, 3 out]
    n152 = call "Camera.vi"("Machine Vision"="Machine Vision 2", "Stop"="Stop", "Camera in"=w308) -> ("Image"=→"Image 2":T2)  [unwired: 2 in, 6 out]
  }
